vi "SMain.vi"() -> ()   [LabVIEW 2011] (continued)
                        n1217 = property on="VISA COM" class="VISAName"() -> ("Text.Text"=w1968:string)  [unwired: 2 in, 2 out]
                        n1218 = local read "Demo"() -> (w1966:bool)
                        n1219 = property on="RS232 I2C Counts" class="VISAName"() -> ("Text.Text"=w1947:string)  [unwired: 2 in, 2 out]
                        n1220 = Build Array(FALSE ("元素"), w1967, w1966, w1965, w1964, w1963, w1952) -> (w1962:bool[])
                        n1221 = property on="打印模式" class="Enum (严格)"() -> ("RingText.Text"=w1955:string)  [unwired: 2 in, 2 out]
                        n1222 = property on="Adaptor:" class="Enum (严格)"() -> ("RingText.Text"=w1954:string)  [unwired: 2 in, 2 out]
                        n1223 = for {
                          tunnel: w1962 -> [w1983] mode=indexing
                          tunnel: [w1980] -> w1960 mode=indexing
                          n1224 = Select(t="TRUE", s=w1983, f="FALSE") -> (s? t:f=w1980:string)
                        }
                        n1225 = local read "upload"() -> (w1976:bool)
                        n1226 = property on="Printer VISA" class="VISAName"() -> ("Text.Text"=w1958:string)  [unwired: 2 in, 2 out]
                        n1227 = property on="RS232 I2C VISA" class="VISAName"() -> ("Text.Text"=w1973:string)  [unwired: 2 in, 2 out]
                        n1228 = Build Array(w1972, w1971, w1970, w1969, w1968) -> (w1961:string[])
                        n1229 = Insert Into Array(array=w1961, new element=w1960) -> (w1959:string[])  [unwired: 1 in]
                        n1230 = Select(t="TRUE", s=w1976, f="FALSE") -> (s? t:f=w1977:string)
                        n1231 = local read "Port Type"() -> (w1978:u16)
                        n1232 = Select(t="TRUE", s=w1949, f="FALSE") -> (s? t:f=w1948:string)
                        n1233 = Number To Decimal String(number=w1978) -> (decimal integer string=w1979:string)  [unwired: 1 in]
                        n1234 = Build Array(w1958, w1973, w1977, w1979, w1955, w1954, w1948, w1947) -> (w1957:string[])
                        n1235 = Insert Into Array(array=w1959, new element=w1957) -> (w1953:string[])  [unwired: 1 in]
                      }
                      frame #1 {
                        n1236 = call <vilib>:"Application Directory.vi"() -> ("Application Directory"=w1989:path)
                        n1237 = Build Path(base path=w1989, name or relative path="database\\initializeConfig.txt" ("名称或相对路径")) -> (appended path=w1986:path)
                        n1238 = call-poly <vilib>:"Read From Spreadsheet File.vi"("file path (dialog if empty)"=w1986) -> ("all rows"=w1988:string[][])  [unwired: 6 in, 4 out]
                        n1239 = Replace Array Subset(array=w1988, new element=w1984, index (col)=1 ("禁用的索引 (列)")) -> (w1985:string[][])  [unwired: 1 in]
                        n1240 = call-poly <vilib>:"Write To Spreadsheet File.vi"("2D data"=w1985, "file path (dialog if empty)"=w1986) -> ()  [unwired: 6 in, 1 out]
                      }
                      frame #2 {
                        n1241 = Wait (ms)(milliseconds to wait=u32 200 ("等待时间（毫秒）")) -> ()  [unwired: 1 out]
                      }
                    }
                  }
                }
              }
              event "打印模式": Value Change {
                n1242 = event-data() -> ("NewVal"=w1992:enum16{"IT Print", "EE Print"})  [unwired: 1 in, 4 out]
                n1243 = case shown="\"IT Print\", 默认" w1992 {
                  frame "IT Print", Default {
                    n1244 = property on="MO:" class="Str"("Visible"=TRUE ("可见")) -> ()  [unwired: 2 in, 2 out]
                    n1245 = local write "EE Write"(TRUE ("EE Write")) -> ()
                  }
                  frame "EE Print" {
                    n1246 = property on="MO:" class="Str"("Visible"=FALSE ("可见")) -> ()  [unwired: 2 in, 2 out]
                  }
                }
              }
              event Panel Close {
                n1247 = event-data() -> ()  [unwired: 1 in, 3 out]
                n1248 = flat-sequence {
                  tunnel: [FALSE ("Stop")] -> w1996
                  frame #0 {
                  }
                  frame #1 {
                  }
                  frame #2 {
                    n1249 = local write "State"("exit" ("state")) -> ()
                  }
                }
              }
              event "Report Type:": Value Change {
                n1250 = event-data() -> ("NewVal"=w2001:u16)  [unwired: 1 in, 4 out]
                n1251 = case shown="1" w2001 {
                  tunnel: [w2002 w2003] -> w2000
                  tunnel: [w2002 w2003] -> w1999
                  frame 0, Default {
                    w2002 = FALSE ("可见")
                  }
                  frame 1 {
                    w2003 = TRUE ("可见")
                  }
                }
                n1252 = property on="Start Page" class="DigNum (严格)"("Visible"=w2000) -> ()  [unwired: 2 in, 2 out]
                n1253 = property on="End Page" class="DigNum (严格)"("Visible"=w1999) -> ()  [unwired: 2 in, 2 out]
              }
              event "VNA VISA": Value Change {
                n1254 = event-data() -> ()  [unwired: 1 in, 5 out]
                n1255 = property on="VNA VISA" class="VISAName"() -> ("Text.Text"=w2004:string)  [unwired: 2 in, 2 out]
                n1256 = Search/Split String(string=w2004, search string/char (-)="N5224A" ("搜索字符串/字符(-)")) -> (offset of match=w2007:i32)  [unwired: 1 in, 2 out]
                n1257 = case shown="-1" w2007 {
                  tunnel: [w2013 0] -> w2006
                  tunnel: [w2012 2] -> w2005
                  tunnel: w2004 -> [w2010 _]
                  frame -1 {
                    n1258 = Search/Split String(string=w2010, search string/char (-)="E5071C" ("搜索字符串/字符(-)")) -> (offset of match=w2009:i32)  [unwired: 1 in, 2 out]
                    n1259 = case shown="-1" w2009 {
                      tunnel: [1 1] -> w2013
                      tunnel: [0 1] -> w2012
                      frame 0..20, Default {
                      }
                      frame -1 {
                      }
                    }
                  }
                  frame 1..20, Default {
                  }
                }
                n1260 = property on="VNA Model:" class="Enum (严格)"("Value"=w2005) -> ()  [unwired: 2 in, 2 out]
                n1261 = property on="Port Type" class="Ring (严格)"("Value"=w2006) -> ()  [unwired: 2 in, 2 out]
              }
              event "VNA Model:": Value Change {
                n1262 = event-data() -> ()  [unwired: 1 in, 5 out]
                n1263 = case shown="\"N5224A\"" "VNA Model:" {
                  tunnel: [u16 1 ("Port Type") u16 1 ("Port Type") u16 0 ("Port Type")] -> w2020
                  frame "E5071C", Default {
                  }
                  frame "N5230A(C)" {
                  }
                  frame "N5224A" {
                  }
                }
                n1264 = property on="Port Type" class="Ring (严格)"("Value"=w2020) -> ()  [unwired: 2 in, 2 out]
              }
              event "Urgent Stop": Value Change {
                n1265 = event-data() -> ("NewVal"=w2025:bool)  [unwired: 1 in, 4 out]
                n1266 = local write "Urgent Stop"(w2025) -> ()
                n1267 = global write "全局.vi" "manual stop"(w2025) -> ()
              }
              event "Manual": Value Change {
                n1268 = event-data() -> ()  [unwired: 1 in, 5 out]
                n1269 = local read "Manual"() -> (w2027:bool)
                n1270 = local read "Demo"() -> (w2026:bool)
                n1271 = local read "DAQ  Model:"() -> (w2030:T14)
                n1272 = local read "DAQ Device"() -> (w2029:u16)
                n1273 = local read "VISA COM"() -> (w2031:refnum<visa-resource-name>)
                n1274 = Or(x=w2027, y=w2026) -> (x .or. y?=w2028:bool)
                n1275 = case shown="假" w2028 {
                  tunnel: w2029 -> [w2034 _]
                  tunnel: w2030 -> [w2033 _]
                  tunnel: w2031 -> [w2032 _]
                  frame False {
                    n1276 = case shown="\"LX MCU\"" w2033 {
                      tunnel: w2034 -> [w2039 _ _]
                      tunnel: w2032 -> [_ w2041 w2043]
                      frame "NI PCI-6509", Default {
                        n1277 = local read "Switch array"() -> (w2037:bool[][])
                        n1278 = call "6509 simple.vi"("error in"="error in 2", "index (row)"=i8 39, "array input: P0-P1-P2-P3-P4-P5"=w2037, "DAQ device"=w2039) -> ("error out"=→"error out 2":errorcluster)  [unwired: 3 in]
                      }
                      frame "LX MCU" {
                        w2040 = u16 1 items=["Testing", "Close All"] ("Function")
                        n1279 = call "MCU Switch Control.vi"("Function"=w2040, "VISA"=w2041) -> ()  [unwired: 9 in, 1 out]
                      }
                      frame "LX MCU_40G" {
                        w2042 = u16 1 items=["Testing", "Close All"] ("Function")
                        n1280 = call "40G MCU Switch Control.vi"("Function"=w2042, "VISA"=w2043) -> ()  [unwired: 9 in, 1 out]
                      }
                    }
                  }
                  frame True {
                  }
                }
              }
              event "DAQ  Model:": Value Change {
                n1281 = event-data() -> ()  [unwired: 1 in, 5 out]
                n1282 = local read "DAQ  Model:"() -> (w2046:T14)
                n1283 = case shown="\"LX MCU_40G\"" w2046 {
                  tunnel: [2 0 0] -> w2045
                  tunnel: [0 2 2] -> w2044
                  frame "NI PCI-6509", Default {
                  }
                  frame "LX MCU" {
                  }
                  frame "LX MCU_40G" {
                  }
                }
                n1284 = property on="DAQ Device" class="Ring (严格)"("DisabledEnum"=w2044) -> ()  [unwired: 2 in, 2 out]
                n1285 = property on="VISA COM" class="VISAName"("DisabledEnum"=w2045) -> ()  [unwired: 2 in, 2 out]
              }
              event Key Down {
                n1286 = event-data() -> ("ScanCode"=w2055:i16)  [unwired: 1 in, 8 out]
                n1287 = disable-structure shown="启用" {
                  frame Disabled {
                    n1288 = call "keyboard_VNA_jet.vi"() -> ()  [unwired: 9 in, 1 out]
                  }
                  frame Enabled {
                  }
                }
                n1289 = local read "midVar_bool_find"() -> (w2057:bool)
                n1290 = Equal?(x=w2055, y=i16 28) -> (x = y?=w2053:bool)
                n1291 = And(x=w2053, y=w2057) -> (x .and. y?=w2056:bool)
                n1292 = case shown="真" w2056 {
                  frame False {
                    n1293 = local write "State"("wait" ("state")) -> ()
                  }
                  frame True {
                    n1294 = flat-sequence {
                      frame #0 {
                        n1295 = property on="P/N:" class="Str"("Key Focus"=FALSE ("键选中")) -> ()  [unwired: 2 in, 2 out]
                      }
                      frame #1 {
                        n1296 = local read "S/N:"() -> (w2061:string)
                        n1297 = Empty String/Path?(string/path=w2061) -> (empty?=w2060:bool)
                        n1298 = case shown="假" w2060 {
                          frame False {
                            n1299 = local write "State"("test" ("state")) -> ()
                          }
                          frame True {
                            n1300 = local write "State"("wait" ("state")) -> ()
                            n1301 = One Button Dialog(message="SN不能为空！") -> ()  [unwired: 1 in, 1 out]
                          }
                        }
                      }
                    }
                  }
                }
              }
              event "Start Test": Value Change {
                n1302 = event-data() -> ()  [unwired: 1 in, 5 out]
                n1303 = local read "midVar_bool_find"() -> (w2065:bool)
                n1304 = case shown="真" w2065 {
                  frame False {
                    n1305 = local write "State"("wait" ("state")) -> ()
                  }
                  frame True {
                    n1306 = local read "S/N:"() -> (w2068:string)
                    n1307 = Empty String/Path?(string/path=w2068) -> (empty?=w2067:bool)
                    n1308 = case shown="假" w2067 {
                      frame False {
                        (unwired) "datacheck" ("State")
                        n1309 = local write "State"("test" ("state")) -> ()
                      }
                      frame True {
                        n1310 = local write "State"("wait" ("state")) -> ()
                        n1311 = One Button Dialog(message="SN不能为空！") -> ()  [unwired: 1 in, 1 out]
                      }
                    }
                  }
                }
              }
              event Menu Selection (User) {
                n1312 = event-data() -> ("MenuRef"=w2075:refnum<k9>, "ItemTag"=w2076:string)  [unwired: 1 in, 4 out]
                n1313 = control-ref of="Test Status:"() -> (w2073:refnum<vi>)
                n1314 = local read "DB1"() -> (w2072:T8)
                n1315 = case shown="\"Project Management\"" w2076 {
                  selector: w2076 -> [_ _ _ _ _ _ _ _ _ _ _ _ w2117 w2130 _]
                  tunnel: w2075 -> [_ _ _ _ _ _ _ _ _ _ _ _ w2116 w2129 _]
                  tunnel: "error in" -> [w2077 _ _ _ _ _ _ _ _ _ _ _ _ _ _]
                  tunnel: w2073 -> [_ _ _ _ _ _ _ _ w2098 _ _ _ _ _ _]
                  tunnel: w2072 -> [_ _ _ w2080 w2089 _ _ _ _ _ _ _ w2113 w2126 _]
                  frame "6509 Switch Tool", Default {
                    n1316 = call "RF Switch tool.vi"("error in"=w2077) -> ("Error out"=→"error out":errorcluster)  [unwired: 6 in]
                  }
                  frame "MCU Switch Tool" {
                    n1317 = local read "DAQ  Model:"() -> (w2079:T14)
                    n1318 = case shown="\"LX MCU_40G_HuaWei\"" w2079 {
                      frame "LX MCU", Default {
                        n1319 = call "RF Switch tool by MCU.vi"() -> ()  [unwired: 8 in]
                      }
                      frame "LX MCU_40G_HuaWei" {
                        n1320 = call "RF Switch tool by MCU HuaWei.vi"() -> ()  [unwired: 8 in]
                      }
                      frame "LX MCU_40G" {
                        n1321 = call "40G RF Switch Matrix.vi"() -> ()  [unwired: 8 in]
                      }
                    }
                  }
                  frame "40G 6509" {
                    n1322 = call "40G RF Switch Tool(NI 6509).vi"() -> ()  [unwired: 8 in]
                  }
                  frame "Project Management" {
                    n1323 = call "LoginForm.vi"("DBSet"=w2080) -> ("厂区"=w2082:string, "登录成功"=w2084:bool, "用户名"=w2083:string)
                    n1324 = local read "DB2"() -> (w2081:T8)
                    n1325 = case shown="真" w2084 {
                      tunnel: w2083 -> [_ w2087]
                      tunnel: w2082 -> [_ w2088]
                      tunnel: w2081 -> [_ w2086]
                      frame False {
                        n1326 = One Button Dialog(message="密码或用户名错误" ("消息")) -> ()  [unwired: 1 in, 1 out]
                      }
                      frame True {
                        n1327 = call "New Project.vi"("DBSet"=w2086, "UserID"=w2087, "厂区"=w2088) -> ()  [unwired: 9 in]
                      }
                    }
                  }
                  frame "SampleImport" {
                    n1328 = call "LoginForm.vi"("DBSet"=w2089) -> ("厂区"=w2091:string, "登录成功"=w2093:bool, "用户名"=w2092:string)
                    n1329 = local read "DB2"() -> (w2090:T8)
                    n1330 = case shown="真" w2093 {
                      tunnel: w2092 -> [_ w2097]
                      tunnel: w2091 -> [_ _]
                      tunnel: w2090 -> [_ _]
                      tunnel: w2089 -> [_ w2096]
                      frame False {
                        n1331 = One Button Dialog(message="密码或用户名错误" ("消息")) -> ()  [unwired: 1 in, 1 out]
                      }
                      frame True {
                        n1332 = local read "SystemMode"() -> (w2095:string)
                        n1333 = call "importNewSample.vi"("DBSet"=w2096, "setNo"=w2095, "user"=w2097) -> ()  [unwired: 9 in]
                      }
                    }
                  }
                  frame "Fixture Management" {
                  }
                  frame "S4P Data Tool" {
                    n1334 = call "S4P Tool.vi"() -> ()  [unwired: 12 in]
                  }
                  frame "EEPROM Editor" {
                    n1335 = call "SubMain2_ChartEEPROM_vna_wmg.vi"() -> ()  [unwired: 12 in]
                  }
                  frame "Label Debug" {
                    n1336 = local read "打印模式"() -> (w2099:enum16{"IT Print", "EE Print"})
                    n1337 = case shown="\"IT Print\", 默认" w2099 {
                      tunnel: w2098 -> [w2107 _]
                      frame "IT Print", Default {
                        n1338 = local read "PRINT"() -> (w2109:refnum<k24>)
                        n1339 = local read "P/N:"() -> (w2108:string)
                        n1340 = local read "DB1"() -> (w2100:T8)
                        n1341 = local read "Fast Print"() -> (w2101:bool)
                        n1342 = local read "SN"() -> (w2110:refnum<k24>)
                        n1343 = property class="Str"(reference=w2107) -> (reference out=w2103:refnum<vi>, "Value"=w2106:string)  [unwired: 1 in, 1 out]
                        n1344 = call "资讯重打标签.vi"("DBSet"=w2100, "print path local"=w2101, "PN"=w2108, "PRINT"=w2109, "SN"=w2110) -> ("PrintMsg"=w2104:string)  [unwired: 6 in]
                        n1345 = Concatenate Strings(w2106, "\n", w2104) -> (w2102:string)
                        n1346 = property class="Str"(reference=w2103, "Value"=w2102) -> ()  [unwired: 1 in, 2 out]
                      }
                      frame "EE Print" {
                        n1347 = call "re-print.vi"() -> ()  [unwired: 12 in]
                      }
                    }
                  }
                  frame "Impedance Test Tool" {
                    n1348 = call "Impedance Testing Tool.vi"() -> ()  [unwired: 12 in]
                  }
                  frame "Control Counting module" {
                    n1349 = call "登录对话框.vi"() -> ("登录状态"=w2111:bool)  [unwired: 3 in, 3 out]
                    n1350 = case shown="真" w2111 {
                      frame False {
                      }
                      frame True {
                        n1351 = local read "RS232 I2C Counts"() -> (w2112:refnum<visa-resource-name>)
                        n1352 = call "初始化使用次数和寿命的界面.vi"("VISA  2"=w2112) -> ()  [unwired: 11 in]
                      }
                    }
                  }
                  frame "Eeprom Write Delay Config" {
                    n1353 = call "saveDelayConfig_烧录.vi"() -> ()  [unwired: 9 in, 3 out]
                  }
                  frame "Excel Data Export" {
                    n1354 = Get Menu Item Info(7:w2117, 11:w2116) -> (0:w2120:errorcluster, 2:w2119:string, 3:w2121:refnum<k9>, 4:w2118:bool)  [unwired: 1 in, 3 out]
                    n1355 = Not(x=w2118) -> (.not. x?=w2115:bool)
                    n1356 = case shown="假" w2115 {
                      selector: w2115 -> [_ w2125]
                      tunnel: [w2124 w2125] -> w2114
                      tunnel: w2113 -> [w2122 _]
                      frame False {
                        n1357 = call "LoginForm.vi"("DBSet"=w2122) -> ("登录成功"=w2123:bool)  [unwired: 2 out]
                        n1358 = Not(x=w2123) -> (.not. x?=w2124:bool)
                      }
                      frame True {
                      }
                    }
                    "Excel?" <- w2114
                    n1359 = Set Menu Item Info(6:w2114, 7:w2117, 8:w2120, 10:w2119, 11:w2121) -> ()  [unwired: 2 in, 2 out]
                  }
                  frame "Data UpLoad" {
                    n1360 = Get Menu Item Info(7:w2130, 11:w2129) -> (0:w2133:errorcluster, 2:w2132:string, 3:w2134:refnum<k9>, 4:w2131:bool)  [unwired: 1 in, 3 out]
                    n1361 = Not(x=w2131) -> (.not. x?=w2128:bool)
                    n1362 = case shown="假" w2128 {
                      selector: w2128 -> [_ w2138]
                      tunnel: [w2137 w2138] -> w2127
                      tunnel: w2126 -> [w2135 _]
                      frame False {
                        n1363 = call "LoginForm.vi"("DBSet"=w2135) -> ("登录成功"=w2136:bool)  [unwired: 2 out]
                        n1364 = Not(x=w2136) -> (.not. x?=w2137:bool)
                      }
                      frame True {
                      }
                    }
                    "upload" <- w2127
                    n1365 = Set Menu Item Info(6:w2127, 7:w2130, 8:w2133, 10:w2132, 11:w2134) -> ()  [unwired: 2 in, 2 out]
                  }
                  frame "Help" {
                    n1366 = call "Help.vi"() -> ()  [unwired: 20 in]
                  }
                }
              }
              event "Type": Value Change {
                n1367 = event-data() -> ()  [unwired: 1 in, 5 out]
                n1368 = local read "SystemMode"() -> (w2149:string)
                n1369 = property on="Type" class="Ring (严格)"() -> ("RingText.Text"=w2145:string)  [unwired: 2 in, 2 out]
                n1370 = Search and Replace String(input string="SELECT goldenSampleNo,caiData FROM cali_sample WHERE setNo='@SystemMode@' AND status='1' and type='@type@'", search string="@SystemMode@" ("搜索字符串"), replace string=w2149) -> (result string=w2147:string)  [unwired: 5 in, 3 out]
                n1371 = Search and Replace String(input string=w2147, search string="@type@" ("搜索字符串"), replace string=w2145) -> (result string=w2144:string)  [unwired: 5 in, 3 out]
                n1372 = local read "DB1"() -> (w2148:T8)
                n1373 = call "query.net.vi"("Sql"=w2144, "DBSet"=w2148) -> ("result"=w2143:string[][])  [unwired: 8 in, 1 out]
                n1374 = Index Array(array=w2143, index (col)=0 ("禁用的索引 (列)")) -> (element=w2141:string[])  [unwired: 1 in]
                n1375 = property on="sampleNo" class="Ring (严格)"("Strings []"=w2141) -> ()  [unwired: 2 in, 2 out]
                n1376 = Array Size(array=w2141) -> (size(s)=w2140:i32)
                n1377 = Greater Than 0?(x=w2140) -> (x > 0?=w2139:bool)
                n1378 = case shown="假" w2139 {
                  frame False {
                    n1379 = property on="sampleNo" class="Ring (严格)"("Val(Sgnl)"=u16 0 ("值(信号)")) -> ()  [unwired: 2 in, 2 out]
                  }
                  frame True {
                    n1380 = property on="sampleNo" class="Ring (严格)"("Val(Sgnl)"=u16 0 ("值(信号)")) -> ()  [unwired: 2 in, 2 out]
                  }
                }
              }
              event "sampleNo": Value Change {
                n1381 = event-data() -> ()  [unwired: 1 in, 5 out]
                n1382 = property on="sampleNo" class="Ring (严格)"() -> ("RingText.Text"=w2163:string)  [unwired: 2 in, 2 out]
                n1383 = Search and Replace String(input string="SELECT caiData FROM cali_sample WHERE goldenSampleNo='@goldenSampleNoe@' AND status='1'", search string="@goldenSampleNoe@" ("搜索字符串"), replace string=w2163) -> (result string=w2162:string)  [unwired: 5 in, 3 out]
                n1384 = local read "DB1"() -> (w2164:T8)
                n1385 = call "query.net.vi"("Sql"=w2162, "DBSet"=w2164) -> ("result"=w2161:string[][])  [unwired: 8 in, 1 out]
                n1386 = Index Array(array=w2161, index (row)=0 ("索引 (行)")) -> (element=w2156:string[])  [unwired: 1 in]
                n1387 = Array Size(array=w2156) -> (size(s)=w2159:i32)
                n1388 = Equal?(x=w2159, y=1) -> (x = y?=w2157:bool)
                n1389 = case shown="真" w2157 {
                  tunnel: w2156 -> [_ w2171]
                  tunnel: [_ w2169] -> w2155
                  tunnel: [FALSE TRUE] -> w2154
                  frame False {
                  }
                  frame True {
                    n1390 = Index Array(array=w2171, index=0 ("索引")) -> (element=w2169:string)
                  }
                }
                "sampleData" <- w2155
                "caliDataSelect" <- w2154
              }
              event "P/N:": Value Change {
                n1391 = event-data() -> ()  [unwired: 1 in, 5 out]
                n1392 = property on="线别" class="Ring (严格)"() -> ("RingText.Text"=w2177:string)  [unwired: 2 in, 2 out]
                n1393 = local read "SystemMode"() -> (w2179:string)
                n1394 = Concatenate Strings("当前线别为：" ("字符串"), w2177, "是否正确" ("字符串")) -> (w2175:string)
                n1395 = Two Button Dialog(message=w2175) -> (T button?=w2174:bool)  [unwired: 2 in]
                "线别确认" <- w2174
                n1396 = local read "DB2"() -> (w2172:T8)
                n1397 = property on="线别" class="Ring (严格)"("DisabledEnum"=T17."Enabled" ("禁用")) -> ()  [unwired: 2 in, 2 out]
                n1398 = case shown="假" w2174 {
                  frame False {
                  }
                  frame True {
                    n1399 = property on="线别" class="Ring (严格)"("DisabledEnum"=T17."Disabled and Grayed Out" ("禁用")) -> ()  [unwired: 2 in, 2 out]
                  }
                }
                n1400 = local write "AutoSN"(FALSE ("AutoSN")) -> ()
                n1401 = local read "Demo"() -> (w2182:bool)
                n1402 = call "Query Project by PN.vi"("Luxshare_P/N:"="P/N:", "System_Mode"=w2179, "Local"="Local Database", "DBSet"=w2172) -> ("Find?"=w2183:bool, "Basic Information"=w2188:string[], "Project  Information"=w2189:string[][], "limitSpec"=w2187:string[][], "SwitchMatrix"=w2186:i32[][], "Label Content"=w2185:string)  [unwired: 9 in, 1 out]
                n1403 = case shown="真" w2183 {
                  tunnel: w2189 -> [_ w2201]
                  tunnel: w2188 -> [_ w2200]
                  tunnel: w2187 -> [_ w2198]
                  tunnel: w2186 -> [_ w2199]
                  tunnel: w2185 -> [_ w2196]
                  tunnel: w2182 -> [_ w2197]
                  tunnel: "P/N:" -> [_ w2195]
                  frame False {
                    w2192 = 2 ("索引")
                    w2193 = "" ("P/N:")
                    n1404 = local write "Sample Description"(w2193) -> ()
                    n1405 = local write "P/N:"(w2193) -> ()
                    n1406 = property on="Start Test" class="Bool"("DisabledEnum"=w2192) -> ()  [unwired: 2 in, 2 out]
                    n1407 = property on="VNA Initial" class="Bool"("DisabledEnum"=w2192) -> ()  [unwired: 2 in, 2 out]
                    n1408 = local write "midVar_bool_find"(FALSE ("midVar_bool_find")) -> ()
                  }
                  frame True {
                    n1409 = global write "全局.vi" "print templete"(TRUE ("print templete")) -> ()
                    n1410 = stacked-sequence {
                      tunnel: w2201 -> [_ _ _ _ _ w2363 _ _ _ _ _ _ _ _ _]
                      tunnel: w2200 -> [_ w2252 w2289 w2295 w2298 _ _ _ _ _ _ _ w2536 _ _]
                      tunnel: w2199 -> [_ _ _ _ _ _ _ _ w2422 _ _ _ _ _ _]
                      tunnel: w2198 -> [_ _ _ _ w2296 w2340 _ _ _ _ _ _ _ _ _]
                      tunnel: w2197 -> [_ _ _ _ _ _ _ _ _ _ w2445 _ _ _ _]
                      tunnel: w2196 -> [_ w2236 _ _ _ _ _ _ _ _ _ _ _ _ _]
                      tunnel: w2195 -> [_ _ _ _ _ _ _ _ _ _ _ w2460 w2530 _ _]
                      frame #0 {
                        n1411 = local read "打印模式"() -> (w2204:enum16{"IT Print", "EE Print"})
                        n1412 = local write "MO Num"(i64 0 ("MO Num")) -> ()
                        n1413 = local write "Pro Num"(i64 0 ("Pro Num")) -> ()
                        n1414 = case shown="\"IT Print\", 默认" w2204 {
                          frame "IT Print", Default {
                            n1415 = local read "MO:"() -> (w2206:string)
                            n1416 = local read "P/N:"() -> (w2210:string)
                            n1417 = local read "SN"() -> (w2207:refnum<k24>)
                            n1418 = local write "EE Write"(TRUE ("EE Write")) -> ()
                            n1419 = call "资讯打标签-检测工单料号匹配.vi"("工单号"=w2206, "料号"=w2210, "引用"=w2207) -> ("工单号、料号检测情况"=w2209:string, "工单数量"=w2208:string)  [unwired: 9 in, 2 out]
                            n1420 = case shown="\"00\", 默认" w2209 {
                              tunnel: w2208 -> [_ _ w2221]
                              tunnel: w2206 -> [_ _ w2220]
                              frame "00", Default {
                                n1421 = local write "midVar_bool_find"(FALSE ("midVar_bool_find")) -> ()
                                n1422 = One Button Dialog(message="工单不存在,输入错误或者线长没有在Tiptop中激活！" ("消息")) -> ()  [unwired: 1 in, 1 out]
                              }
                              frame "10" {
                                n1423 = local write "midVar_bool_find"(FALSE ("midVar_bool_find")) -> ()
                                n1424 = One Button Dialog(message="工单存在，和料号不匹配！" ("消息")) -> ()  [unwired: 1 in, 1 out]
                              }
                              frame "11" {
                                n1425 = Decimal String To Number(string=w2221) -> (number=w2222:i32)  [unwired: 2 in, 1 out]
                                n1426 = String Subset(string=w2220, length (rest)=5 ("长度（剩余）")) -> (substring=w2218:string)  [unwired: 1 in]
                                n1427 = To Upper Case(1:w2218) -> (0:w2217:string)
                                n1428 = local write "MO Num"(w2222) -> ()
                                n1429 = Equal?(x=w2217, y="E511D") -> (x = y?=w2215:bool)
                                "正常工单?" <- w2215
                                n1430 = case shown="假" w2215 {
                                frame False {
                                n1431 = One Button Dialog(message="不是正常工单号，如测试的是华为料号，\n将不会上传数据到华为，请注意！") -> ()  [unwired: 1 in, 1 out]
                                }
                                frame True {
                                }
                                }
                                n1432 = local write "midVar_bool_find"(TRUE ("midVar_bool_find")) -> ()
                              }
                            }
                          }
                          frame "EE Print" {
                            n1433 = call <vilib>:"Application Directory.vi"() -> ("Application Directory"=w2228:path)
                            n1434 = local read "P/N:"() -> (w2229:string)
                            n1435 = Build Path(base path=w2228, name or relative path="Database\\FigoConfig.xml") -> (appended path=w2226:path)
                            n1436 = call "EEWriteJudge.vi"("path to XML document"=w2226, "PN"=w2229) -> ("Write?"=w2225:bool)  [unwired: 9 in]
                            "EE Write" <- w2225
                            n1437 = local write "midVar_bool_find"(TRUE ("midVar_bool_find")) -> ()
                            n1438 = case shown="假" w2225 {
                              frame False {
                                n1439 = One Button Dialog(message="EE模式不进行烧录") -> ()  [unwired: 1 in, 1 out]
                              }
                              frame True {
                              }
                            }
                          }
                        }
                      }
                      frame #1 {
                        (unwired) "LuxsharePN,CustomerPN,Customer,SampleDes,AWG,Length,EEPROMWrite,LabelPrint,Remarks" ("查询项目")
                        n1440 = call "littleVI_2_part#LabelStr.vi"("input_label"=w2236) -> ("show_label"=→"Label Type":string[])  [unwired: 10 in]
                        n1441 = Index Array(array=w2252, index #1=3 ("索引"), index #2=4 ("索引"), index #3=5 ("索引"), index #4=2 ("索引")) -> (element #1=w2241:string, element #2=w2240:string, element #3=w2239:string, element #4=→"CustomerName":string)
                        "Length" <- w2239
                        n1442 = call "littleVI_1_DesString.vi"("input_Length"=w2239, "input_AWG"=w2240, "input_sampleDes"=w2241) -> ("PNDes"=→"PN Des":string, "SampleDes"=w2238:string)  [unwired: 7 in]
                        n1443 = local write "midVar_bool_find"(TRUE ("midVar_bool_find")) -> ()
                        n1444 = property on="Start Test" class="Bool"("DisabledEnum"=2 ("索引")) -> ()  [unwired: 2 in, 2 out]
                        n1445 = property on="Sample Description" class="Str"("Value"=w2238, "Visible"=TRUE ("可见")) -> ()  [unwired: 2 in, 2 out]
                        n1446 = property on="Result" class="Str"("Visible"=FALSE ("可见"), "Value"="Testing..." ("Result"), "DisabledEnum"=1, "Text.BGColor"=u32 16777216) -> ()  [unwired: 2 in, 2 out]
                        n1447 = local write "labelConfig"(string[] [] ("labelConfig")) -> ()
                      }
                      frame #2 {
                        w2270 = "" ("元素")
                        # "CusPN"
                        # "AWG"
                        n1448 = Index Array(array=w2289, index #1=1 ("索引"), index #2=2 ("索引"), index #3=4 ("索引"), index #4=6 ("索引"), index #8=11 ("索引")) -> (element #1=w2262:string, element #2=→"Cus":string, element #3=w2271:string, element #4=w2287:string, element #5=w2283:string, element #6=w2280:string, element #7=w2277:string, element #8=w2259:string, element #9=w2258:string)  [unwired: 4 in]
                        n1449 = local read "P/N:"() -> (w2274:string)
                        n1450 = call <vilib>:"Trim Whitespace.vi"("string"=w2287) -> ("trimmed string"=w2286:string)  [unwired: 1 in]
                        n1451 = call <vilib>:"Trim Whitespace.vi"("string"=w2259) -> ("trimmed string"=w2268:string)  [unwired: 1 in]
                        n1452 = call <vilib>:"Trim Whitespace.vi"("string"=w2280) -> ("trimmed string"=w2279:string)  [unwired: 1 in]
                        n1453 = call <vilib>:"Trim Whitespace.vi"("string"=w2277) -> ("trimmed string"=w2276:string)  [unwired: 1 in]
                        n1454 = Spreadsheet String To Array(delimiter (Tab)="," ("分隔符(Tab)"), format string="" ("格式字符串"), spreadsheet string=w2258, array type (2D Dbl)=string[] []) -> (array=w2263:string[])
                        n1455 = call <vilib>:"Trim Whitespace.vi"("string"=w2283) -> ("trimmed string"=→"FixtureNo":string)  [unwired: 1 in]
                        n1456 = Equal?(x=w2268, y="1") -> (x = y?=w2257:bool)
                        "AutoSN" <- w2257
                        n1457 = Equal?(x=w2286, y="1") -> (x = y?=→"EEPROMTF":bool)
                        n1458 = Equal?(x=w2279, y="1") -> (x = y?=→"LabelTF":bool)
                        n1459 = Decimal String To Number(string=w2276) -> (number=→"LabelNum":i32)  [unwired: 2 in, 1 out]
                        n1460 = Build Array(w2274, w2271, w2270, w2270, w2262) -> (w2253:string[])
                        "Data In" <- w2253
                        n1461 = local write "frePoints"(w2263) -> ()
                        n1462 = Index Array(array=w2253, index=4 ("索引")) -> (element=w2254:string)
                        n1463 = call <vilib>:"Trim Whitespace.vi"("string"=w2254) -> ("trimmed string"=→"customerPN":string)  [unwired: 1 in]
                        n1464 = case shown="真" w2257 {
                          frame False {
                            n1465 = local write "S/N:"("" ("S/N:")) -> ()
                            n1466 = property on="S/N:" class="Str"("DisabledEnum"=T17."Enabled" ("禁用")) -> ()  [unwired: 2 in, 2 out]
                          }
                          frame True {
                            n1467 = local write "S/N:"("automatic sn" ("S/N:")) -> ()
                            n1468 = property on="S/N:" class="Str"("DisabledEnum"=T17."Disabled and Grayed Out" ("禁用")) -> ()  [unwired: 2 in, 2 out]
                          }
                        }
                      }
                      frame #3 {
                        n1469 = local read "Local Database"() -> (w2294:bool)
                        n1470 = case shown="真" w2294 {
                          tunnel: w2295 -> [_ _]
                          frame False {
                          }
                          frame True {
                          }
                        }
                      }
                      frame #4 {
                        (unwired) FALSE
                        n1471 = local read "EEPROMTF"() -> (w2299:bool)
                        n1472 = local read "Local Database"() -> (w2297:bool)
                        n1473 = case shown="真" w2299 {
                          tunnel: w2298 -> [_ w2301]
                          tunnel: w2297 -> [_ w2300]
                          frame False {
                          }
                          frame True {
                            n1474 = case shown="假" w2300 {
                              tunnel: w2301 -> [_ w2330]
                              frame False {
                                # "此处的mid_array_eep是已经拓展OK的"
                                n1475 = local read "DB2"() -> (w2303:T8)
                                n1476 = local read "DB1"() -> (w2304:T8)
                                n1477 = local read "P/N:"() -> (w2318:string)
                                n1478 = call "getDataFromSQL.vi"("DB"=w2304, "input_str_PN"=w2318) -> ("DateCode8Format_0X30"=w2306:string, "show_str_labelType"=w2313:string, "show_array_eep"=w2315:string[][], "show_bool_valid"=w2316:bool, "show_bool_exsit"=w2317:bool, "show_str_message"=w2314:string, "PN description"=→"PN description":string)  [unwired: 1 out]
                                n1479 = call "boolsToString.vi"("input_bool_low"=w2316, "input_bool_high"=w2317) -> ("show_str_01string"=w2319:string)
                                n1480 = local write "mid_str_labelType"(w2313) -> ()
                                n1481 = call "getLabelConfigFromSQL.vi"("input_str_labelType"=w2313, "DB"=w2303) -> ("show_array"=w2307:string[])
                                n1482 = local write "mid_array_eep"(w2315) -> ()
                                n1483 = case shown="\"10\"" w2319 {
                                tunnel: w2314 -> [w2322 w2325 _]
                                tunnel: [2 ("索引") 2 ("索引") 0 ("索引")] -> w2308
                                frame "00", "01", Default {
                                n1484 = One Button Dialog(message=w2322) -> ()  [unwired: 1 in, 1 out]
                                n1485 = local write "midVar_bool_find"(FALSE ("midVar_bool_find")) -> ()
                                }
                                frame "10" {
                                n1486 = One Button Dialog(message=w2325) -> ()  [unwired: 1 in, 1 out]
                                n1487 = local write "midVar_bool_find"(FALSE ("midVar_bool_find")) -> ()
                                }
                                frame "11" {
                                n1488 = local write "midVar_bool_find"(TRUE ("midVar_bool_find")) -> ()
                                }
                                }
                                n1489 = Decimal String To Number(string=w2306) -> (number=→"DateCode8Value_0X30":i32)  [unwired: 2 in, 1 out]
                                n1490 = Index Array(array=w2307, index #1=0 ("索引"), index #2=11 ("索引")) -> (element #1=w2309:string, element #2=w2310:string)
                                n1491 = local write "mid_str_snformat"(w2310) -> ()
                                n1492 = local write "labelConfig"(w2307) -> ()
                                n1493 = local write "mid_str_descrip"(w2309) -> ()
                                n1494 = property on="Start Test" class="Bool"("DisabledEnum"=w2308) -> ()  [unwired: 2 in, 2 out]
                                n1495 = property on="VNA Initial" class="Bool"("DisabledEnum"=w2308) -> ()  [unwired: 2 in, 2 out]
                              }
                              frame True {
                                n1496 = Index Array(array=w2330, index #1=13 ("索引"), index #2=14 ("索引")) -> (element #1=w2329:string, element #2=w2332:string)
                                n1497 = local read "P/N:"() -> (w2335:string)
                                n1498 = local write "mid_str_snformat"(w2332) -> ()
                                n1499 = local write "mid_str_labelType"(w2329) -> ()
                                n1500 = call "littleVI_4_readLocalEEPROMFile.vi"("input_PN"=w2335) -> ("show_eeprom"=w2334:string[][])  [unwired: 10 in]
                                n1501 = local write "mid_str_descrip"("" ("mid_str_descrip")) -> ()
                                n1502 = local write "mid_array_eep"(w2334) -> ()
                              }
                            }
                          }
                        }
                        "limitSpec" <- w2296
                      }
                      frame #5 {
                        n1503 = call "Detailed Project Information.vi"("Project  Information Input"=w2363) -> ("TDR Setting2"=→"TDR Setting  2":string[], "minus 2X?"=w2350:bool, "CMP Setting"=w2345:string[], "smooth point"=w2339:i32, "TDR Test Item Name"=→"TDR Test Item Name":string[], "Report Config"=→"Report Config":string[], "ILD Spec No"=→"ILD Spec No":i32, "Report Name"=→"Report Temp. Name":string, "S-para Pair Name"=→"S-para Pair Name":string[], "TDR Setting"=→"TDR Setting":string[], "NEXT Pair Name"=→"NEXT Pair Name":string[], "FEXT Pair Name"=→"FEXT Pair Name":string[], "Diff Test Item Name"=w2348:string[], "Spec Association Col No"=w2354:string[], "Cal File Path"=w2360:string[])  [unwired: 11 in, 1 out]
                        "Spec Association Col No" <- w2354
                        "smooth point" <- w2339
                        "Diff Test Item smooth" <- w2348
                        n1504 = local write "Dem 2X"(w2350) -> ()
                        n1505 = Index Array(array=w2360, index=0 ("索引")) -> (element=→"Cal File Path":string)
                        n1506 = for {
                          tunnel: w2348 -> [w2373] mode=indexing
                          tunnel: [w2370] -> w2342 mode=indexing
                          tunnel: [w2367] -> w2341 mode=indexing
                          n1507 = Search and Replace String(input string=w2373, search string=",smooth" ("搜索字符串"), replace string="" ("替换字符串(\"\")")) -> (result string=w2370:string, number of replacements=w2368:i32)  [unwired: 5 in, 2 out]
                          n1508 = Equal?(x=w2368, y=1) -> (x = y?=w2367:bool)
                        }
                        "Diff Test Item Name" <- w2342
                        n1509 = Decimal String To Number(string=w2354) -> (number=→"Spec _Col":i32[])  [unwired: 2 in, 1 out]
                        n1510 = control-ref of="Tab_Graph"() -> (w2366:refnum<vi>)
                        n1511 = call "Tap Title Modflication.vi"("Test Item Name"=w2348, "Tab_Graph"=w2366) -> ()  [unwired: 10 in]
                        n1512 = call "TestItemCount.vi"("Testitems"=w2348) -> ("Count"=→"Count":i16)
                        n1513 = Index Array(array=w2345, index=0 ("索引")) -> (element=→"CMP setting":string)
                        n1514 = call "Divide Test Items.vi"("Test Item Name"=w2342) -> ("Crosstalk  Item List"=→"Crosstalk Item List":string[], "S-Para Item List"=→"S-Para Item List":string[])  [unwired: 9 in]
                        n1515 = call "getSparaConfig.vi"("Spec Associate"=w2340, "different"=w2342, "smooth"=w2341, "smoothPoints"=w2339) -> ("sPara"=w2338:T3[], "extPara"=w2337:T3[])  [unwired: 10 in]
                        n1516 = Insert Into Array(array=w2338, new element=w2337) -> (→"sSpec":T3[])  [unwired: 1 in]
                      }
                      frame #6 {
                        n1517 = local read "TDR Setting"() -> (w2397:string[])
                        n1518 = Index Array(array=w2397) -> (element #1=w2396:string, element #2=w2395:string, element #3=w2394:string, element #4=w2393:string, element #5=w2391:string, element #6=w2390:string, element #7=w2389:string, element #8=→"Fix Delay(ns)":string, element #9=w2379:string, element #10=w2382:string)  [unwired: 10 in]
                        n1519 = Decimal String To Number(string=w2379) -> (number=→"Skew Spec(ps)":i32)  [unwired: 2 in, 1 out]
                        n1520 = Fract/Exp String To Number(string=w2395) -> (number=w2386:dbl)  [unwired: 3 in, 1 out]
                        n1521 = Fract/Exp String To Number(string=w2396) -> (number=w2387:dbl)  [unwired: 3 in, 1 out]
                        n1522 = Decimal String To Number(string=w2394) -> (number=w2385:i32)  [unwired: 2 in, 1 out]
                        n1523 = Spreadsheet String To Array(format string="%s" ("格式字符串"), spreadsheet string=w2382, array type (2D Dbl)=dbl[] []) -> (array=→"2X IL":dbl[])  [unwired: 1 in]
                        n1524 = Fract/Exp String To Number(string=w2393) -> (number=w2376:dbl)  [unwired: 3 in, 1 out]
                        n1525 = Equal?(x=w2390, y="1") -> (x = y?=w2388:bool)
                        n1526 = Fract/Exp String To Number(string=w2391) -> (number=w2384:dbl)  [unwired: 3 in, 1 out]
                        n1527 = local write "Impedance Spec String"(w2389) -> ()
                        n1528 = local write "Start TimeNs"(w2387) -> ()
                        n1529 = local write "StopTimeNs"(w2386) -> ()
                        n1530 = local write "Data Points"(w2385) -> ()
                        n1531 = local write "Filter Risetime(ps)"(w2376) -> ()
                        n1532 = local write "Compensation(ohm)"(w2384) -> ()
                        n1533 = local write "Impedance Filter"(w2388) -> ()
                        n1534 = Greater?(x=w2376, y=65.0) -> (0:w2374:bool)
                        n1535 = case shown="真" w2374 {
                          frame False {
                          }
                          frame True {
                            n1536 = One Button Dialog(message="risetime时间大于65，请联系钟波\n或方羽确认是否正确！") -> ()  [unwired: 1 in, 1 out]
                          }
                        }
                      }
                      frame #7 {
                        n1537 = local read "TDR Setting  2"() -> (w2420:string[])
                        n1538 = Index Array(array=w2420) -> (element #1=w2419:string, element #2=w2418:string, element #3=w2417:string, element #4=w2416:string, element #5=w2414:string, element #6=w2413:string, element #7=w2412:string, element #8=→"Fix Delay(ns)  2":string, element #9=w2401:string, element #10=w2404:string)  [unwired: 10 in]
                        n1539 = Decimal String To Number(string=w2401) -> (number=→"Skew Spec(ps) 2":i32)  [unwired: 2 in, 1 out]